vi "2_VisualizeModulePositioning2-Backup.vi"(0 "Placement Monitor":T1(plugin-control)=refnum, 1 "Calibrated positions of fiducials [mm]":dbl[][](array[numeric])=[[-658.867386146, 115.937184375, -18.342965965], [-563.38738772, 115.95451918, -18.342965965], [-563.369748267, 18.796520782, -18.342965965], [-658.849746693, 18.779185977, -18.342965965], [-560.867387761, 115.954976697, -18.342965965], [-465.387389335, 115.972311502, -18.342965965], [-465.369749882, 18.814313103, -18.342965965], [-560.849748308, 18.796978298, -18.342965965], [-462.867389377, 115.972769019, -18.342965965], [-367.38739095, 115.990103824, -18.342965965], [-367.369751497, 18.832105425, -18.342965965], [-462.849749923, 18.81477062, -18.342965965], [-364.867390992, 115.990561341, -18.342965965], [-269.387392565, 116.007896146, -18.342965965], [-269.369753112, 18.849897747, -18.342965965], [-364.849751539, 18.832562942, -18.342965965], [-266.867392607, 116.008353663, -18.342965965], [-171.38739418, 116.025688468, -18.342965965], [-171.369754727, 18.867690069, -18.342965965], [-266.849753154, 18.850355264, -18.342965965], [-168.867394222, 116.026145985, -18.342965965], [-73.387395796, 116.04348079, -18.342965965], [-73.369756342, 18.885482391, -18.342965965], [-168.849754769, 18.868147586, -18.342965965], [-70.867395837, 116.043938306, -18.342965965], [24.612602589, 116.061273111, -18.342965965], [24.630242042, 18.903274713, -18.342965965], [-70.849756384, 18.885939908, -18.342965965], [27.132602548, 116.061730628, -18.342965965], [122.612600974, 116.079065433, -18.342965965], [122.630240427, 18.921067035, -18.342965965], [27.150242001, 18.90373223, -18.342965965], [125.132600933, 116.07952295, -18.342965965], [220.612599359, 116.096857755, -18.342965965], [220.630238812, 18.938859356, -18.342965965], [125.150240386, 18.921524551, -18.342965965], [223.132599318, 116.097315272, -18.342965965], [318.612597744, 116.114650077, -18.342965965], [318.630237197, 18.956651678, -18.342965965], [223.150238771, 18.939316873, -18.342965965], [321.132597702, 116.115107594, -18.342965965], [416.612596129, 116.132442399, -18.342965965], [416.630235582, 18.974444, -18.342965965], [321.150237156, 18.957109195, -18.342965965], [419.132596087, 116.132899916, -18.342965965], [514.612594514, 116.150234721, -18.342965965], [514.630233967, 18.992236322, -18.342965965], [419.15023554, 18.974901517, -18.342965965], [517.132594472, 116.150692238, -18.342965965], [612.612592899, 116.168027043, -18.342965965], [612.630232352, 19.010028644, -18.342965965], [517.150233925, 18.992693839, -18.342965965]], 2 "XYZ .NET Refnum in":refnum<k24>, 3 "Axis Speeds":T10={"X [mm/s]"=25.0, "Y [mm/s]"=25.0, "Z [mm/s]"=25.0}, 4 "Module fiducial marker":T7=enum."Mark C", 5 "N modules":i32=13, 6 "Sensor Pattern":T8(ring)=enum."ATLAS12", 7 "error in (no error)":errorcluster, 8 "Templates path":path=path "C:/Users/Aerotech/Documents/BNL_ThermomechanicalStave", 9 "Calibration [um/pix]":dbl=1.55, 10 "Current Build Phase":refnum<vi>, 11 "Temperature":refnum<vi>, 12 "Module #":refnum<vi>, 13 "Placement tolerance [um]":dbl=25.0, 14 "Tape Type":T5=enum."Axial (Sutcliffe NP49-01-100 01-Mar-16)", 16 "Module Report":refnum<vi>, 17 "Base notes":string, 18 "Reports path":path=path "C:/Users/Aerotech/cernbox/BNL/Stave Assembly Records/2017-05-15/ModulePlacement") -> (19 "Recalibrated??":bool, 22 "XYZ .NET Refnum out":refnum<k24>, 27 "error out":errorcluster)   [LabVIEW 2016]
uses:
  Utils/Controls/All_Enums/Enum_TypeDef_FidMarkers.ctl
  C:/Users/Aerotech/Documents/BNLStaveAssembly-blueprint/Bin/Aerotech.A3200.dll
  BNLStaveAssembly-blueprint/Bin/Aerotech.A3200.dll
  Utils/Controls/All_Enums/Enum_TypeDef_CornerSelection.ctl
  Utils/Controls/All_Enums/Enum_TypeDef_TapeType.ctl
panel:
  out "Order":string[](array[string])
  out "Templates":T1[](array[plugin-control])
  out "Fiducial Template 2":T1(plugin-control)
  in  "Recalibrate!!":bool
  in  "Exit to survey or glue":bool
  out "Current task:":string="Applying glue for Module 11"
  in  "Tab Control: Positioning and Surveys":T2(tab)=enum."Apply glue"
  out "Offset interpreter":T3={"Offset Interpreter - Right"=FALSE, "Offset Interpreter - forward"=FALSE, "Offset Interpreter - backward"=TRUE, "Offset Interpreter - Left"=TRUE, "Placement Confirmation"=FALSE}
  in  "User Report: Current Module":T4={"B"=FALSE, "A"=FALSE, "D"=FALSE, "C"=FALSE, "ID"="", "Module #"=11, "x, centre"=368.8814166421462, "y, centre"=67.54477579693595, "Aligned"=FALSE, "Glue applied"=FALSE, "Placed"=FALSE}
  out "X offset [um]":sgl=497.0423
  out "Y offset [um]":sgl=417.2712
  in  "Module corner loop stop":bool
  in  "Center-only search?":bool
  in  "User notes":string="Type your note here...."
  out "Module # str":string="Module 11"
  in  "Assembly step":string(combo)
  in  "Manual Z?":bool
  in  "Manual Z [mm]":dbl
  in  "Dots (T) or Lines (F)":bool
  in  "Send XYZ Stage Away":bool
  in  "Work on Corner...":T6=enum."[Exit]"
  in  "Work on Module #...":i32=11
  in  "Tab Control":enum32{"Fiducial marker", "Error reporting"}(tab)
  out "Fiducial Template":T1(plugin-control)
  out "Mark string":string="MarkC"
  out "Current Stage Position":T9={"X [mm]"=416.6304080435383, "Y [mm]"=18.974446486493466, "Z [mm]"=-18.342965704975803}
  out "Module Progress Report":T11(array[cluster])=[{"B"=FALSE, "A"=FALSE, "D"=FALSE, "C"=FALSE, "ID"="", "Module #"=1, "x, centre"=-611.1185672065, "y, centre"=67.3668525785, "Aligned"=FALSE, "Glue applied"=FALSE, "Placed"=FALSE}, {"B"=FALSE, "A"=FALSE, "D"=FALSE, "C"=FALSE, "ID"="", "Module #"=2, "x, centre"=-513.1185688215, "y, centre"=67.3846449, "Aligned"=FALSE, "Glue applied"=FALSE, "Placed"=FALSE}, {"B"=FALSE, "A"=FALSE, "D"=FALSE, "C"=FALSE, "ID"="", "Module #"=3, "x, centre"=-415.118570437, "y, centre"=67.402437222, "Aligned"=FALSE, "Glue applied"=FALSE, "Placed"=FALSE}, {"B"=FALSE, "A"=FALSE, "D"=FALSE, "C"=FALSE, "ID"="", "Module #"=4, "x, centre"=-317.118572052, "y, centre"=67.420229544, "Aligned"=FALSE, "Glue applied"=FALSE, "Placed"=FALSE}, {"B"=FALSE, "A"=FALSE, "D"=FALSE, "C"=FALSE, "ID"="", "Module #"=5, "x, centre"=-219.118573667, "y, centre"=67.438021866, "Aligned"=FALSE, "Glue applied"=FALSE, "Placed"=FALSE}, {"B"=FALSE, "A"=FALSE, "D"=FALSE, "C"=FALSE, "ID"="", "Module #"=6, "x, centre"=-121.118575282, "y, centre"=67.455814188, "Aligned"=FALSE, "Glue applied"=FALSE, "Placed"=FALSE}, {"B"=FALSE, "A"=FALSE, "D"=FALSE, "C"=FALSE, "ID"="", "Module #"=7, "x, centre"=-23.118576897500002, "y, centre"=67.4736065095, "Aligned"=FALSE, "Glue applied"=FALSE, "Placed"=FALSE}, {"B"=FALSE, "A"=FALSE, "D"=FALSE, "C"=FALSE, "ID"="", "Module #"=8, "x, centre"=74.8814214875, "y, centre"=67.4913988315, "Aligned"=FALSE, "Glue applied"=FALSE, "Placed"=FALSE}, {"B"=FALSE, "A"=FALSE, "D"=FALSE, "C"=FALSE, "ID"="", "Module #"=9, "x, centre"=172.8814198725, "y, centre"=67.509191153, "Aligned"=FALSE, "Glue applied"=FALSE, "Placed"=FALSE}, {"B"=FALSE, "A"=FALSE, "D"=FALSE, "C"=FALSE, "ID"="", "Module #"=10, "x, centre"=270.8814182575, "y, centre"=67.52698347500001, "Aligned"=FALSE, "Glue applied"=FALSE, "Placed"=FALSE}, {"B"=FALSE, "A"=FALSE, "D"=FALSE, "C"=FALSE, "ID"="", "Module #"=11, "x, centre"=368.8814166421462, "y, centre"=67.54477579693595, "Aligned"=FALSE, "Glue applied"=FALSE, "Placed"=FALSE}, {"B"=FALSE, "A"=FALSE, "D"=FALSE, "C"=FALSE, "ID"="", "Module #"=12, "x, centre"=466.881415027, "y, centre"=67.562568119, "Aligned"=FALSE, "Glue applied"=FALSE, "Placed"=FALSE}, {"B"=FALSE, "A"=FALSE, "D"=FALSE, "C"=FALSE, "ID"="", "Module #"=13, "x, centre"=564.881413412, "y, centre"=67.580360441, "Aligned"=FALSE, "Glue applied"=FALSE, "Placed"=FALSE}]
  # "VISUALIZE MODULE PLACEMENT Brandeis University - Brookhaven National Laboratory * ATLAS Phase II Inner Tracker Upgrade * Primary Authors: Hannah Herde (hherde@brandeis.edu), Laura Bergsten (lbergsten@brandeis.edu)"
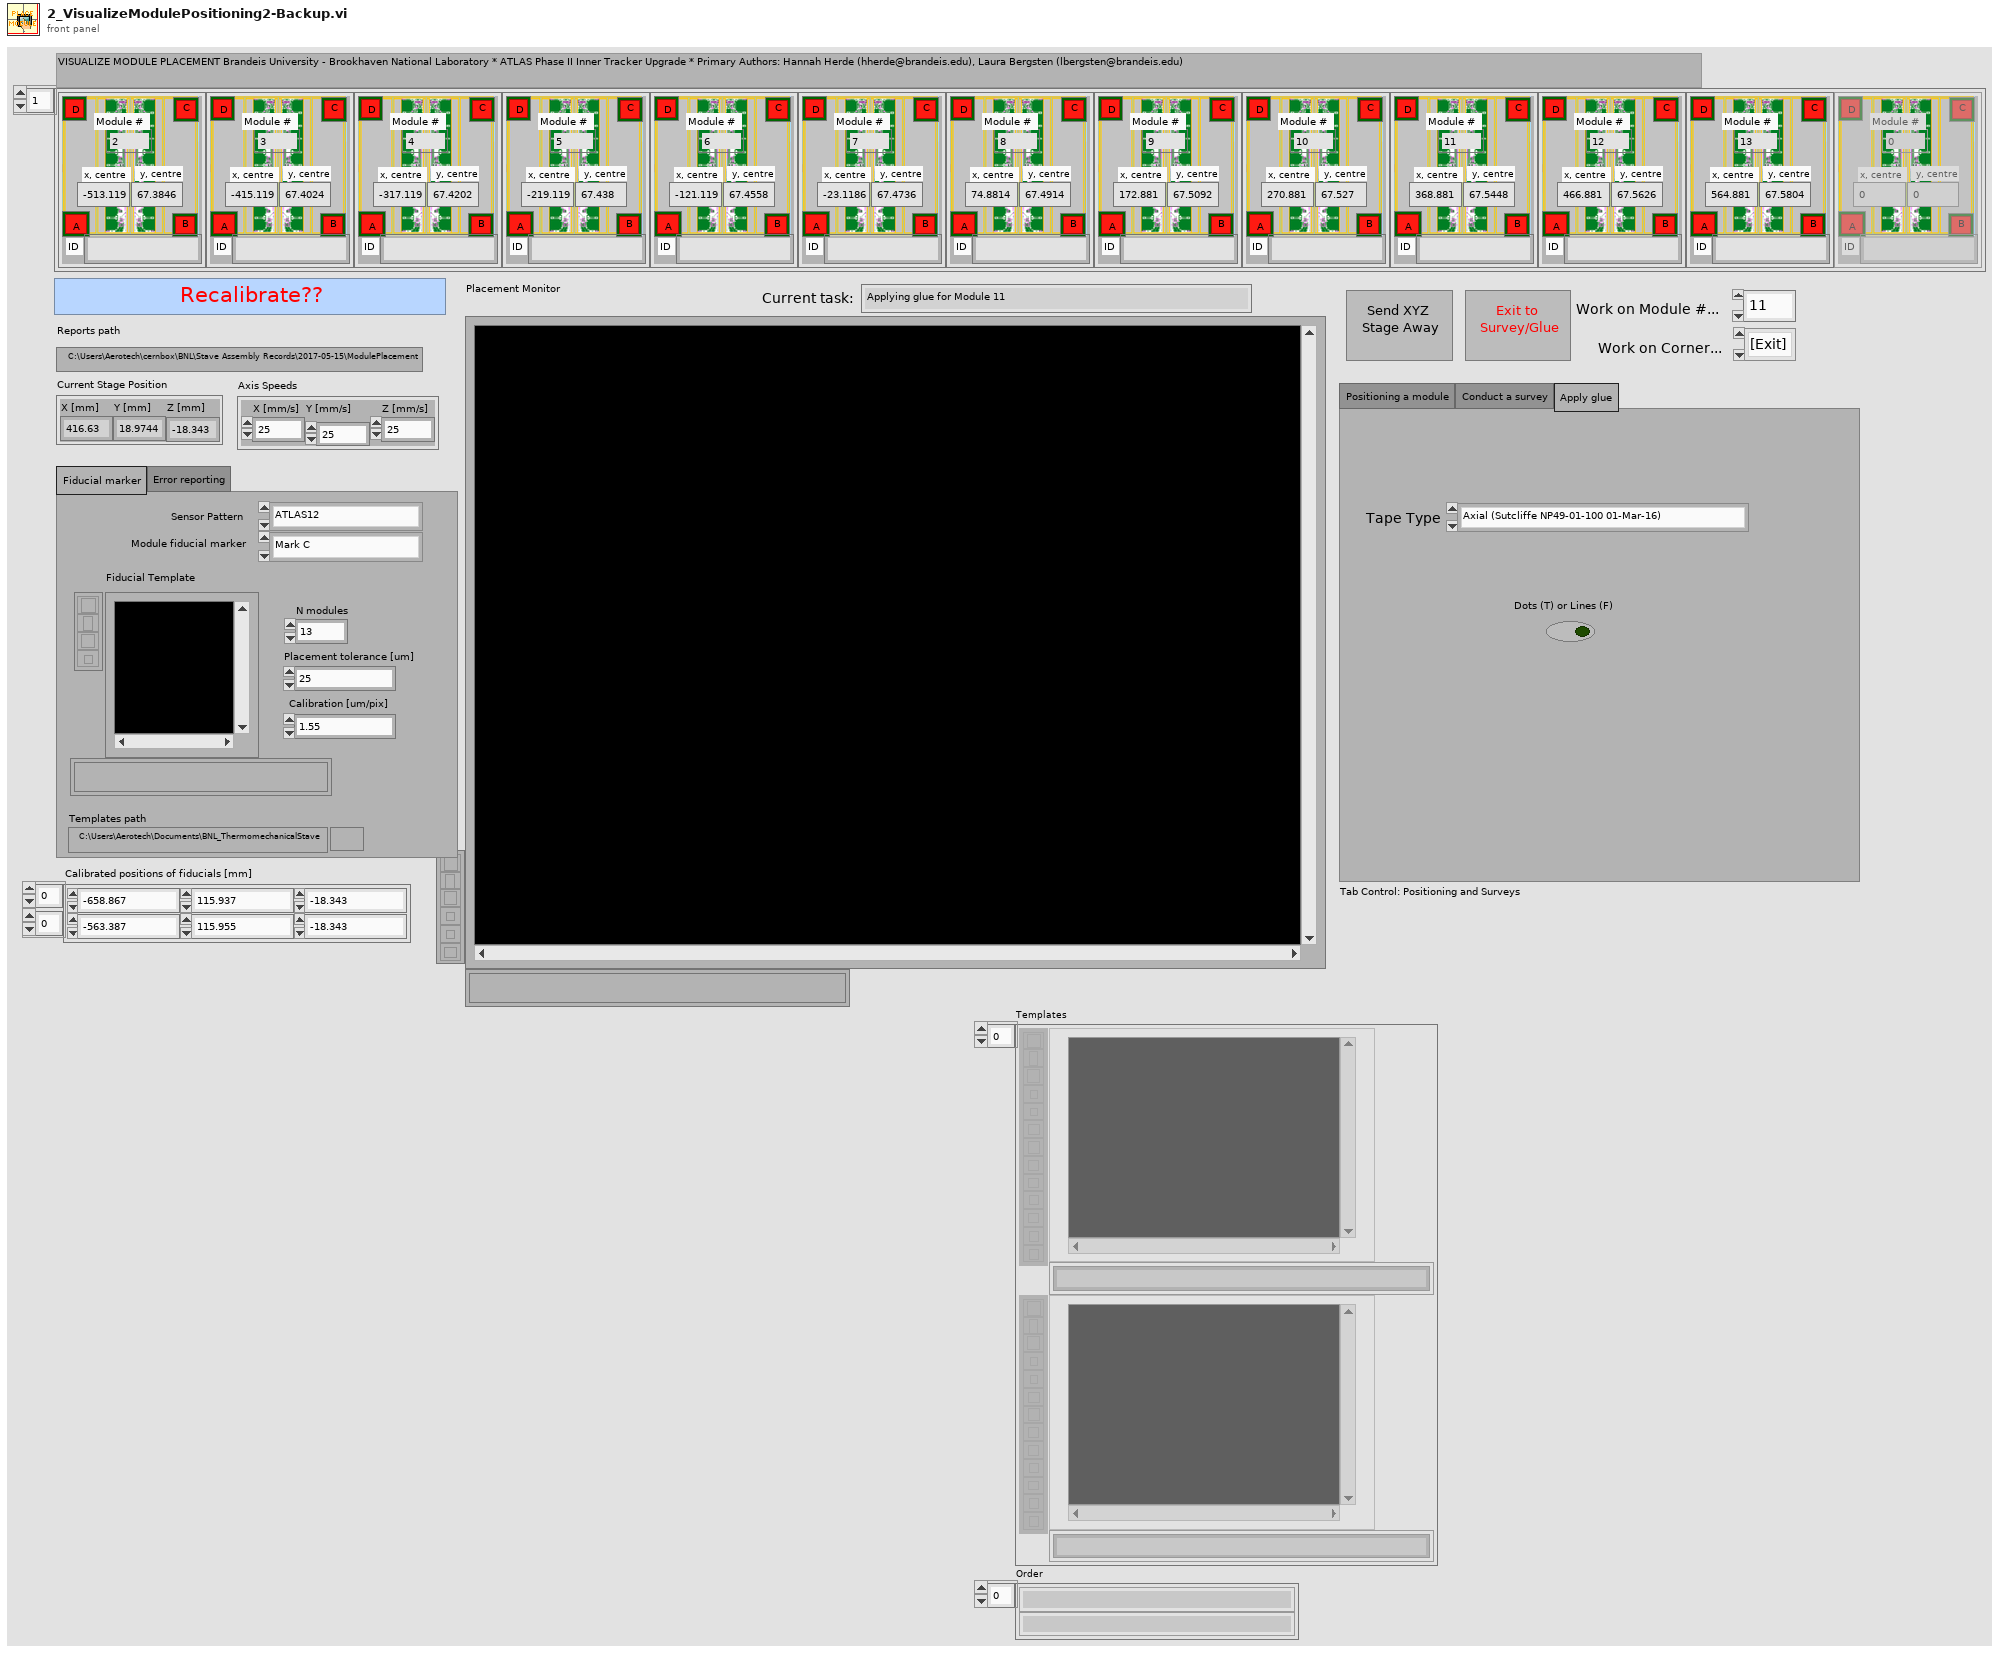
[diagram p1: front panel]
types:
  T1 = typedef "IMAQ Image.ctl" = refnum<image>
  T2 = enum32{"Positioning a module", "Conduct a survey", "Apply glue"}
  T3 = cluster{"Offset Interpreter - Right":bool, "Offset Interpreter - forward":bool, "Offset Interpreter - backward":bool, "Offset Interpreter - Left":bool, "Placement Confirmation":bool}
  T4 = cluster{"B":bool, "A":bool, "D":bool, "C":bool, "ID":string, "Module #":i32, "x, centre":dbl, "y, centre":dbl, "Aligned":bool, "Glue applied":bool, "Placed":bool}
  T5 = typedef "Enum_TypeDef_TapeType.ctl" = enum16{"Right stereo", "Left stereo", "Stereo (Sutcliffe NP49-01-100 01-Mar-16)", "Stereo (Sutcliffe 21-Jun-18- Electrical)", "Axial (Sutcliffe NP49-01-100 01-Mar-16)"}
  T6 = typedef "Enum_TypeDef_CornerSelection.ctl" = enum16{"A", "B", "C", "D", "[Exit]"}
  T7 = typedef "Enum_TypeDef_FidMarkers.ctl" = enum16{"Mark B", "Mark C", "Bias Ring Corner", "Mark I (Slim/17)", "Mark E (Slim/17)", "Mark F (Slim/17)", "Mark G (Slim/17)", "Mark A (12)", "Kapton Spacers"}
  T8 = enum16{"ATLAS07", "ATLAS12", "ATLAS12Slim", "ATLAS17LS"}
  T9 = cluster{"X [mm]":dbl, "Y [mm]":dbl, "Z [mm]":dbl}
  T10 = cluster{"X [mm/s]":dbl, "Y [mm/s]":dbl, "Z [mm/s]":dbl}
  T11 = cluster{"B":bool, "A":bool, "D":bool, "C":bool, "ID":string, "Module #":i32, "x, centre":dbl, "y, centre":dbl, "Aligned":bool, "Glue applied":bool, "Placed":bool}[]
  T12 = enum8{"Enabled", "Disabled", "Disabled and Grayed Out"}
  T13 = enum16{"Left Button", "Center Button", "Right Button", "Window Close"}
  T14 = cluster{"Final X":dbl, "Final Y":dbl, "Final Z":dbl}
  T15 = cluster{"ID":string, "Mark string":string, "Assembly step":string, "User notes":string, string, "Corner surveyed position":dbl[]}
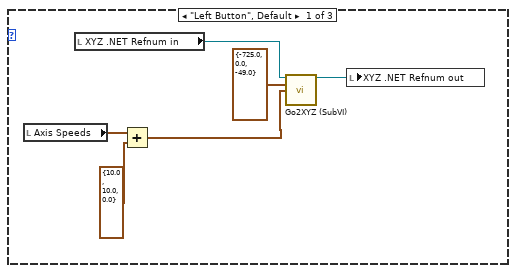
[diagram p3: hidden frame]
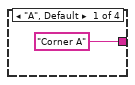
[diagram p6: hidden frame]
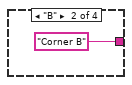
[diagram p7: hidden frame]
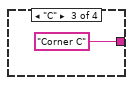
[diagram p8: hidden frame]
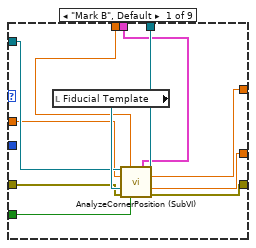
[diagram p9: hidden frame]
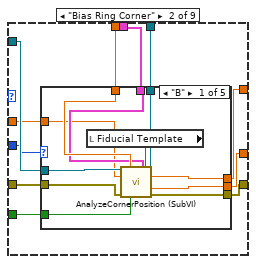
[diagram p10: hidden frame]
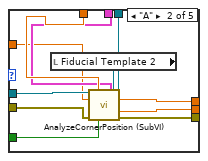
[diagram p11: hidden frame]
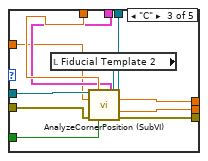
[diagram p12: hidden frame]
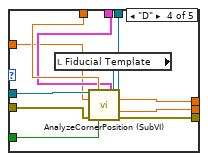
[diagram p13: hidden frame]
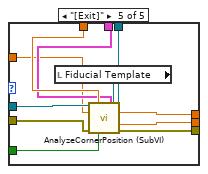
[diagram p14: hidden frame]
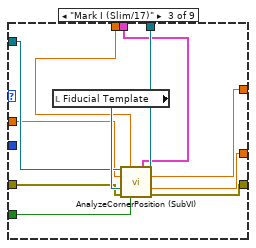
[diagram p15: hidden frame]
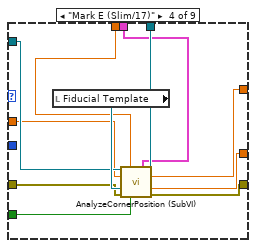
[diagram p16: hidden frame]
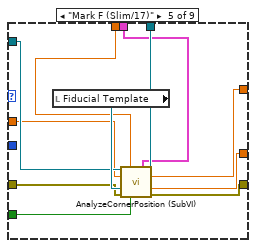
[diagram p17: hidden frame]
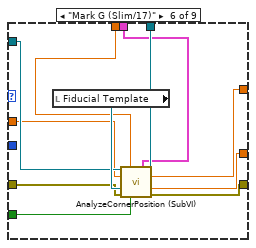
[diagram p18: hidden frame]
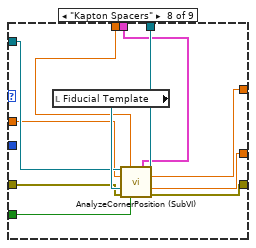
[diagram p19: hidden frame]
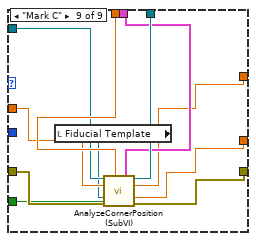
[diagram p20: hidden frame]
diagram:
  n1 = property on="Module corner loop stop" class="Bool"(error in="error in (no error)", "BoolText.Text"="Preparing..." ("Boolean Text.Text"), "DisabledEnum"=T12."Disabled and Grayed Out" ("Disabled")) -> (error out=w14:errorcluster)  [unwired: 1 in, 1 out]
  n2 = call "GetFiducialMarkTemplate (SubVI).vi"("error in (no error)"=w14, "Module fiducial marker"="Module fiducial marker", "Sensor Pattern"="Sensor Pattern", "Templates path"="Templates path") -> ("error out"=w18:errorcluster, "BiasRingCorner"=→"Fiducial Template 2":T1, "Mark string"=w3:string, "Templates"=→"Templates":T1[], "Order"=→"Order":string[])  [unwired: 3 in]
  "Mark string" <- w3
  n3 = for "Generate module placement monitor" {
    N: "N modules" -> [_]
    tunnel: "Calibrated positions of fiducials [mm]" -> [w50]
    tunnel: [w49] -> w12 mode=indexing
    tunnel: w14 -> [w30]
    tunnel: [w38] -> w5 mode=indexing
    tunnel: w3 -> [w34]
    i -> [w33]
    n4 = local read "Reports path"() -> (w32:path)
    n5 = local read "Module Progress Report"() -> (w45:T11)
    n6 = Increment(x=w33) -> (x+1=w28:i32)
    n7 = call "RecursiveDirectoryStructureGenerator (SubVI).vi"("error in (no error)"=w30, "Folder index"=w28, "Host directory"=w32) -> ("error out"=w29:errorcluster, "Nth subfolder in host directory"=w31:path)  [unwired: 7 in]
    n8 = Number To Decimal String(number=w28) -> (decimal integer string=w43:string)  [unwired: 1 in]
    n9 = Concatenate Strings("Module_" ("string"), w43, ".txt" ("string")) -> (w41:string)
    n10 = call "GetModuleReport (SubVI).vi"("error in (no error)"=w29, "Calibrated positions of fiducials [mm]"=w50, "ith Module"=w33, "Module Progress Report in"=w45) -> ("error out"=w47:errorcluster, "MyCorners"=w39:dbl[][], "Array of ith module cluster fiducial mark positions"=w49:cluster{"X":dbl, "Y":dbl, "Z":dbl}[], "Module Progress Report out"=w48:T11)  [unwired: 4 in]
    n11 = property class="Ctl"(reference="Module Report", error in=w47, "Value"=w48) -> (error out=w37:errorcluster)  [unwired: 1 out]
    n12 = Build Path(base path=w31, name or relative path=w41) -> (appended path=w35:path)
    n13 = local write "Module Progress Report"(w48) -> ()
    n14 = for {
      tunnel: string[] ["CornerA", "CornerB", "CornerC", "CornerD"] -> [w59] mode=indexing
      tunnel: w39 -> [w58] mode=indexing
      tunnel: [w57] -> w38
      tunnel: w37 -> [w56]
      tunnel: TRUE ("Write to file") -> [w55]
      tunnel: w35 -> [w54]
      tunnel: w34 -> [w53]
      n15 = call "WriteModuleToFile (SubVI).vi"("Mark used for tracking"=w53, "Assembly step"="Ideal", "User notes"="Base notes", "Current corner"=w59, "Fiducial Mark Position"=w58, "error in (no error)"=w56, "Module reports file path"=w54, "Write to file"=w55) -> ("error out"=w57:errorcluster)  [unwired: 11 in]
    }
  }
  n16 = property on="Fiducial Template" class="ImageControl"(error in=w18, "Zoom to Fit Mode"=TRUE) -> (error out=w11:errorcluster)  [unwired: 1 in, 1 out]
  n17 = property on="Module corner loop stop" class="Bool"(error in=w11, "BoolText.Text"="Preparing..." ("Boolean Text.Text"), "DisabledEnum"=T12."Disabled and Grayed Out" ("Disabled")) -> (error out=w6:errorcluster)  [unwired: 1 in, 1 out]
  n18 = Merge Errors(w6, w5) -> (w8:errorcluster)
  n19 = while {
    stop <- w60 stop-if-true
    n20 = case shown="True" "Send XYZ Stage Away" {
      frame False {
      }
      frame True {
        n21 = flat-sequence {
          frame #0 {
            n22 = call <vilib>:"Three Button Dialog.vi"("Window Title (\"\")"="Move Stage?" ("Window Title (\"\")"), "Right Button Text (\"Cancel\")"="Cancel" ("Assembly step"), "Center Button Text (\"No\")"="RIGHT" ("Assembly step"), "Left Button Text (\"Yes\")"="LEFT" ("Assembly step"), "message"="Be gone XYZ Stage" ("Assembly step")) -> ("Which Button?"=w63:T13)  [unwired: 6 in]
            n23 = case shown="\"Center Button\"" w63 {
              frame "Left Button", Default {
                n24 = local read "Axis Speeds"() -> (w70:T10)
                n25 = local read "XYZ .NET Refnum in"() -> (w73:refnum<k24>)
                n26 = Add(x=w70, y=T10 {"X [mm/s]"=10.0, "Y [mm/s]"=10.0, "Z [mm/s]"=0.0}) -> (x+y=w68:T10)
                n27 = call "Go2XYZ (SubVI).vi"(".NET Refnum in"=w73, "Go to Coordinates"=cluster{"X":dbl, "Y":dbl, "Z":dbl} {"X"=-725.0, "Y"=0.0, "Z"=-49.0}, "Axis Speeds"=w68) -> (".NET Refnum out"=w72:refnum<k24>)  [unwired: 8 in, 4 out]
                n28 = local write "XYZ .NET Refnum out"(w72) -> ()
              }
              frame "Center Button" {
                n29 = local read "Axis Speeds"() -> (w76:T10)
                n30 = local read "XYZ .NET Refnum in"() -> (w78:refnum<k24>)
                n31 = Add(x=w76, y=T10 {"X [mm/s]"=10.0, "Y [mm/s]"=10.0, "Z [mm/s]"=0.0}) -> (x+y=w74:T10)
                n32 = call "Go2XYZ (SubVI).vi"(".NET Refnum in"=w78, "Go to Coordinates"=cluster{"X":dbl, "Y":dbl, "Z":dbl} {"X"=725.0, "Y"=0.0, "Z"=-49.0}, "Axis Speeds"=w74) -> (".NET Refnum out"=w79:refnum<k24>)  [unwired: 8 in, 4 out]
                n33 = local write "XYZ .NET Refnum out"(w79) -> ()
              }
              frame "Right Button" {
              }
            }
          }
          frame #1 {
            n34 = local write "Send XYZ Stage Away"(FALSE) -> ()
          }
        }
      }
    }
    n35 = local read "Recalibrate!!"() -> (w60:bool)
  }
  n36 = while {
    tunnel: w12 -> [w93]
    shift-right: [w90] -> w7
    shift-left: w8 -> [w92]
    stop <- w87 stop-if-true
    # "Align, apply glue, and survey modules"
    n37 = local read "Recalibrate!!"() -> (w87:bool)
    "Recalibrated??" <- w87
    n38 = flat-sequence {
      tunnel: w93 -> [w99]
      tunnel: w92 -> [w97]
      tunnel: [w98] -> w91
      tunnel: [w96] -> w89
      tunnel: w87 -> [w95]
      tunnel: [w94] -> w88
      tunnel: [w393] -> w86
      tunnel: w91 -> [w393]
      tunnel: w89 -> [w392]
      tunnel: [w392] -> w84
      tunnel: w88 -> [w391]
      tunnel: [w390] -> w82
      tunnel: w86 -> [w408]
      tunnel: [w408] -> w85
      tunnel: w84 -> [w407]
      tunnel: [w407] -> w83
      tunnel: w82 -> [w406]
      tunnel: [w406] -> w81
      tunnel: w85 -> [w412]
      tunnel: [w411] -> w90
      tunnel: w83 -> [w410]
      tunnel: w81 -> [w409]
      frame #0 {
        n39 = while {
          tunnel: w99 -> [w107]
          tunnel: [w106] -> w98
          shift-right: [w104] -> w96
          shift-left: w97 -> [w103]
          tunnel: w95 -> [_]
          stop <- w102 stop-if-true
          # "Select module and corner to align"
          n40 = local read "Recalibrate!!"() -> (w101:bool)
          n41 = Equal?(x="Work on Corner...", y=enum16{"A", "B", "C", "D", "[Exit]"}."[Exit]") -> (x = y?=w110:bool)
          n42 = Or(x="Exit to survey or glue", y=w101) -> (x .or. y?=w102:bool)
          n43 = Decrement(x="Work on Module #...") -> (x-1=w108:i32)
          n44 = case shown="False" w110 {
            tunnel: "Work on Corner..." -> [w131 _]
            tunnel: w108 -> [w129 w366]
            tunnel: w107 -> [w127 w367]
            tunnel: [w121 w367] -> w106
            tunnel: "Work on Module #..." -> [w120 _]
            tunnel: w103 -> [w119 w365]
            tunnel: [w115 w363] -> w104
            frame False {
              # "Align modules"
              n45 = flat-sequence {
                tunnel: w131 -> [w132]
                tunnel: [w132] -> w130
                tunnel: w129 -> [w139]
                tunnel: [w140] -> w128
                tunnel: w127 -> [w140]
                tunnel: [w139] -> w126
                tunnel: w120 -> [w138]
                tunnel: w119 -> [w137]
                tunnel: [w136] -> w118
                tunnel: [w132] -> w113
                tunnel: w130 -> [w174]
                tunnel: w128 -> [w172]
                tunnel: w126 -> [w173]
                tunnel: [w173] -> w124
                tunnel: [w172] -> w122
                tunnel: w118 -> [w171]
                tunnel: [w170] -> w117
                tunnel: [w169] -> w114
                tunnel: w113 -> [w169]
                tunnel: [w182] -> w125
                tunnel: w124 -> [w182]
                tunnel: [w181] -> w123
                tunnel: w122 -> [w181]
                tunnel: w117 -> [w180]
                tunnel: [w179] -> w116
                tunnel: w114 -> [w178]
                tunnel: w125 -> [w357]
                tunnel: w123 -> [w356]
                tunnel: [w356] -> w121
                tunnel: w116 -> [w355]
                tunnel: [w354] -> w115
                frame #0 {
                  # "Generate labels"
                  n46 = local read "Module Progress Report"() -> (w142:T11)
                  n47 = case shown="\"D\"" w132 {
                    tunnel: ["Corner A" "Corner B" "Corner C" "Corner D"] -> w155
                    frame "A", Default {
                    }
                    frame "B" {
                    }
                    frame "C" {
                    }
                    frame "D" {
                    }
                  }
                  n48 = Empty String/Path?(string/path="Assembly step") -> (empty?=w135:bool)
                  n49 = case shown="True" w135 {
                    tunnel: [w160 "Working on" ("Assembly step")] -> w133
                    tunnel: "Assembly step" -> [w160 _]
                    frame False {
                    }
                    frame True {
                    }
                  }
                  n50 = Number To Decimal String(number=w138) -> (decimal integer string=w150:string)  [unwired: 1 in]
                  n51 = Index Array(array=w142, index=w139) -> (element=w141:T4)
                  n52 = Concatenate Strings("Module " ("string"), w150) -> (w156:string)
                  "Module # str" <- w156
                  n53 = local write "User Report: Current Module"(w141) -> ()
                  n54 = Concatenate Strings("Done with " ("string"), w156, ",  " ("string"), w155) -> (w154:string)
                  n55 = property on="Module corner loop stop" class="Bool"(error in=w137, "BoolText.Text"=w154, "DisabledEnum"=T12."Enabled" ("Disabled")) -> (error out=w159:errorcluster)  [unwired: 1 in, 1 out]
                  n56 = local read "Module Report"() -> (w143:refnum<vi>)
                  n57 = property class="Str"(reference="Module #", "Value"=w156) -> (error out=w147:errorcluster)  [unwired: 1 in, 1 out]
                  n58 = Concatenate Strings(w133, ": " ("string"), w156) -> (w148:string)
                  n59 = property class="Ctl"(reference=w143, "Value"=w142) -> (error out=w158:errorcluster)  [unwired: 1 in, 1 out]
                  n60 = property class="Str"(reference="Current Build Phase", error in=w147, "Value"=w148) -> (error out=w157:errorcluster)  [unwired: 1 out]
                  n61 = Merge Errors(w158, w157, w159) -> (w136:errorcluster)
                }
                frame #1 {
                  # "Send stage to the corner, or send it out of the way"
                  n62 = Index Array "Select a corner\non a module"(array=w172, index (row)=w173, index (col)=w174) -> (element=w167:cluster{"X":dbl, "Y":dbl, "Z":dbl})
                  n63 = call "Go2XYZ (SubVI).vi"(".NET Refnum in"="XYZ .NET Refnum in", "Go to Coordinates"=w167, "Axis Speeds"="Axis Speeds", "error in (no error)"=w171) -> (".NET Refnum out"=→"XYZ .NET Refnum out":refnum<k24>, "Final Position"=→"Current Stage Position":T14, "error out"=w170:errorcluster)  [unwired: 7 in, 2 out]
                }
                frame #2 {
                  # "Align the corner"
                  n64 = case shown="False" FALSE {
                    tunnel: w180 -> [w185 w353]
                    tunnel: [w184 w353] -> w179
                    tunnel: w178 -> [w183 _]
                    frame False {
                      n65 = while "Module Corner Placement Loop" {
                        shift-right: [w197] -> w184
                        shift-left: w185 -> [w189]
                        tunnel: w183 -> [w187]
                        stop <- "Module corner loop stop" stop-if-true
                        # "Module Corner Alignment Loop"
                        n66 = local read "Module fiducial marker"() -> (w186:T7)
                        n67 = case shown="\"Mark A (12)\"" w186 {
                          tunnel: [w207 w219 w284 w295 w306 w317 w328 w339 w352] -> w197
                          tunnel: [w203 w215 w280 w291 w302 w313 w324 w335 w351] -> w196
                          tunnel: "Placement tolerance [um]" -> [w202 w214 w279 w290 w301 w312 w323 w334 w350]
                          tunnel: "Placement Monitor" -> [w204 w216 w281 w292 w303 w314 w325 w336 w349]
                          tunnel: "Calibration [um/pix]" -> [w200 w212 w277 w288 w299 w310 w321 w332 w348]
                          tunnel: [w201 w213 w278 w289 w300 w311 w322 w333 w347] -> w192
                          tunnel: [w205 w217 w282 w293 w304 w315 w326 w337 w346] -> w191
                          tunnel: [w206 w218 w283 w294 w305 w316 w327 w338 w345] -> w190
                          tunnel: w189 -> [w208 w220 w285 w296 w307 w318 w329 w340 w344]
                          tunnel: "Center-only search?" -> [w199 w211 w276 w287 w298 w309 w320 w331 w343]
                          tunnel: w187 -> [_ w210 _ _ _ _ _ _ _]
                          frame "Mark B", Default {
                            n68 = local read "Fiducial Template"() -> (w209:T1)
                            n69 = call "AnalyzeCornerPosition (SubVI).vi"("Refnum in"=w204, "Placement tolerance [um]"=w202, "Calibration [um/pix]"=w200, "Fiducial Template"=w209, "error in (no error)"=w208, "Center-only search?"=w199) -> ("Offset interpreter"=w201:T3, "Refnum out"=w203:T1, "X offset [um]"=w205:sgl, "Y offset [um]"=w206:sgl, "error out"=w207:errorcluster)  [unwired: 3 in, 2 out]
                          }
                          frame "Bias Ring Corner" {
                            n70 = case shown="\"B\"" w210 {
                              tunnel: w220 -> [w230 w241 w252 w263 w274]
                              tunnel: [w229 w240 w251 w262 w273] -> w219
                              tunnel: [w228 w239 w250 w261 w272] -> w218
                              tunnel: [w227 w238 w249 w260 w271] -> w217
                              tunnel: w216 -> [w226 w237 w248 w259 w270]
                              tunnel: [w225 w236 w247 w258 w269] -> w215
                              tunnel: w214 -> [w224 w235 w246 w257 w268]
                              tunnel: [w223 w234 w245 w256 w267] -> w213
                              tunnel: w212 -> [w222 w233 w244 w255 w266]
                              tunnel: w211 -> [w221 w232 w243 w254 w265]
                              frame "B" {
                                n71 = local read "Fiducial Template"() -> (w231:T1)
                                n72 = call "AnalyzeCornerPosition (SubVI).vi"("Refnum in"=w226, "Placement tolerance [um]"=w224, "Calibration [um/pix]"=w222, "Fiducial Template"=w231, "error in (no error)"=w230, "Center-only search?"=w221) -> ("Offset interpreter"=w223:T3, "Refnum out"=w225:T1, "X offset [um]"=w227:sgl, "Y offset [um]"=w228:sgl, "error out"=w229:errorcluster)  [unwired: 3 in, 2 out]
                              }
                              frame "A" {
                                n73 = local read "Fiducial Template 2"() -> (w242:T1)
                                n74 = call "AnalyzeCornerPosition (SubVI).vi"("Refnum in"=w237, "Placement tolerance [um]"=w235, "Calibration [um/pix]"=w233, "Fiducial Template"=w242, "error in (no error)"=w241, "Center-only search?"=w232) -> ("Offset interpreter"=w234:T3, "Refnum out"=w236:T1, "X offset [um]"=w238:sgl, "Y offset [um]"=w239:sgl, "error out"=w240:errorcluster)  [unwired: 3 in, 2 out]
                              }
                              frame "C" {
                                n75 = local read "Fiducial Template 2"() -> (w253:T1)
                                n76 = call "AnalyzeCornerPosition (SubVI).vi"("Refnum in"=w248, "Placement tolerance [um]"=w246, "Calibration [um/pix]"=w244, "Fiducial Template"=w253, "error in (no error)"=w252, "Center-only search?"=w243) -> ("Offset interpreter"=w245:T3, "Refnum out"=w247:T1, "X offset [um]"=w249:sgl, "Y offset [um]"=w250:sgl, "error out"=w251:errorcluster)  [unwired: 3 in, 2 out]
                              }
                              frame "D" {
                                n77 = local read "Fiducial Template"() -> (w264:T1)
                                n78 = call "AnalyzeCornerPosition (SubVI).vi"("Refnum in"=w259, "Placement tolerance [um]"=w257, "Calibration [um/pix]"=w255, "Fiducial Template"=w264, "error in (no error)"=w263, "Center-only search?"=w254) -> ("Offset interpreter"=w256:T3, "Refnum out"=w258:T1, "X offset [um]"=w260:sgl, "Y offset [um]"=w261:sgl, "error out"=w262:errorcluster)  [unwired: 3 in, 2 out]
                              }
                              frame "[Exit]" {
                                n79 = local read "Fiducial Template"() -> (w275:T1)
                                n80 = call "AnalyzeCornerPosition (SubVI).vi"("Refnum in"=w270, "Placement tolerance [um]"=w268, "Calibration [um/pix]"=w266, "Fiducial Template"=w275, "error in (no error)"=w274, "Center-only search?"=w265) -> ("Offset interpreter"=w267:T3, "Refnum out"=w269:T1, "X offset [um]"=w271:sgl, "Y offset [um]"=w272:sgl, "error out"=w273:errorcluster)  [unwired: 3 in, 2 out]
                              }
                            }
                          }
                          frame "Mark I (Slim/17)" {
                            n81 = local read "Fiducial Template"() -> (w286:T1)
                            n82 = call "AnalyzeCornerPosition (SubVI).vi"("Refnum in"=w281, "Placement tolerance [um]"=w279, "Calibration [um/pix]"=w277, "Fiducial Template"=w286, "error in (no error)"=w285, "Center-only search?"=w276) -> ("Offset interpreter"=w278:T3, "Refnum out"=w280:T1, "X offset [um]"=w282:sgl, "Y offset [um]"=w283:sgl, "error out"=w284:errorcluster)  [unwired: 3 in, 2 out]
                          }
                          frame "Mark E (Slim/17)" {
                            n83 = local read "Fiducial Template"() -> (w297:T1)
                            n84 = call "AnalyzeCornerPosition (SubVI).vi"("Refnum in"=w292, "Placement tolerance [um]"=w290, "Calibration [um/pix]"=w288, "Fiducial Template"=w297, "error in (no error)"=w296, "Center-only search?"=w287) -> ("Offset interpreter"=w289:T3, "Refnum out"=w291:T1, "X offset [um]"=w293:sgl, "Y offset [um]"=w294:sgl, "error out"=w295:errorcluster)  [unwired: 3 in, 2 out]
                          }
                          frame "Mark F (Slim/17)" {
                            n85 = local read "Fiducial Template"() -> (w308:T1)
                            n86 = call "AnalyzeCornerPosition (SubVI).vi"("Refnum in"=w303, "Placement tolerance [um]"=w301, "Calibration [um/pix]"=w299, "Fiducial Template"=w308, "error in (no error)"=w307, "Center-only search?"=w298) -> ("Offset interpreter"=w300:T3, "Refnum out"=w302:T1, "X offset [um]"=w304:sgl, "Y offset [um]"=w305:sgl, "error out"=w306:errorcluster)  [unwired: 3 in, 2 out]
                          }
                          frame "Mark G (Slim/17)" {
                            n87 = local read "Fiducial Template"() -> (w319:T1)
                            n88 = call "AnalyzeCornerPosition (SubVI).vi"("Refnum in"=w314, "Placement tolerance [um]"=w312, "Calibration [um/pix]"=w310, "Fiducial Template"=w319, "error in (no error)"=w318, "Center-only search?"=w309) -> ("Offset interpreter"=w311:T3, "Refnum out"=w313:T1, "X offset [um]"=w315:sgl, "Y offset [um]"=w316:sgl, "error out"=w317:errorcluster)  [unwired: 3 in, 2 out]
                          }
                          frame "Mark A (12)" {
                            n89 = local read "Fiducial Template"() -> (w330:T1)
                            n90 = call "AnalyzeCornerPosition (SubVI).vi"("Refnum in"=w325, "Placement tolerance [um]"=w323, "Calibration [um/pix]"=w321, "Fiducial Template"=w330, "error in (no error)"=w329, "Center-only search?"=w320) -> ("Offset interpreter"=w322:T3, "Refnum out"=w324:T1, "X offset [um]"=w326:sgl, "Y offset [um]"=w327:sgl, "error out"=w328:errorcluster)  [unwired: 3 in, 2 out]
                          }
                          frame "Kapton Spacers" {
                            n91 = local read "Fiducial Template"() -> (w341:T1)
                            n92 = call "AnalyzeCornerPosition (SubVI).vi"("Refnum in"=w336, "Placement tolerance [um]"=w334, "Calibration [um/pix]"=w332, "Fiducial Template"=w341, "error in (no error)"=w340, "Center-only search?"=w331) -> ("Offset interpreter"=w333:T3, "Refnum out"=w335:T1, "X offset [um]"=w337:sgl, "Y offset [um]"=w338:sgl, "error out"=w339:errorcluster)  [unwired: 3 in, 2 out]
                          }
                          frame "Mark C" {
                            n93 = local read "Fiducial Template"() -> (w342:T1)
                            n94 = call "AnalyzeCornerPosition (SubVI).vi"("Refnum in"=w349, "Placement tolerance [um]"=w350, "Calibration [um/pix]"=w348, "Fiducial Template"=w342, "error in (no error)"=w344, "Center-only search?"=w343) -> ("Offset interpreter"=w347:T3, "Refnum out"=w351:T1, "X offset [um]"=w346:sgl, "Y offset [um]"=w345:sgl, "error out"=w352:errorcluster)  [unwired: 3 in, 2 out]
                          }
                        }
                        "X offset [um]" <- w191
                        "Y offset [um]" <- w190
                        "Offset interpreter" <- w192
                        n95 = local write "Placement Monitor"(w196) -> ()
                      }
                    }
                    frame True {
                    }
                  }
                }
                frame #3 {
                  # "Update the module progress report"
                  n96 = local read "Module Progress Report"() -> (w358:T11)
                  n97 = local read "Module Report"() -> (w361:refnum<vi>)
                  n98 = Replace Array Subset(array=w358, new element="User Report: Current Module", index=w357) -> (w359:T11)
                  n99 = property class="Ctl"(reference=w361, error in=w355, "Value"=w359) -> (error out=w354:errorcluster)  [unwired: 1 out]
                  n100 = local write "Module Progress Report"(w359) -> ()
                }
              }
            }
            frame True {
              # "Exit module alignment to do a survey or apply glue"
              n101 = disable-structure shown="Disabled" {
                disable-tunnel: w366 -> [w373 _]
                disable-tunnel: w365 -> [w369 w379]
                disable-tunnel: [w368 w378] -> w364
                frame Disabled {
                  n102 = local read "User Report: Current Module"() -> (w377:T4)
                  n103 = local read "Module Progress Report"() -> (w374:T11)
                  n104 = local read "Module Report"() -> (w376:refnum<vi>)
                  n105 = Replace Array Subset(array=w374, new element=w377, index=w373) -> (w375:T11)
                  n106 = property class="Ctl"(reference=w376, error in=w369, "Value"=w375) -> (error out=w370:errorcluster)  [unwired: 1 out]
                  n107 = local write "Module Progress Report"(w375) -> ()
                  n108 = property on="Module corner loop stop" class="Bool"(error in=w370, "BoolText.Text"="Waiting..." ("Boolean Text.Text"), "DisabledEnum"=T12."Disabled and Grayed Out" ("Disabled")) -> (error out=w368:errorcluster)  [unwired: 1 in, 1 out]
                }
                frame Enabled {
                  n109 = property on="Module corner loop stop" class="Bool"(error in=w379, "BoolText.Text"="Waiting..." ("Boolean Text.Text"), "DisabledEnum"=T12."Disabled and Grayed Out" ("Disabled")) -> (error out=w378:errorcluster)  [unwired: 1 in, 1 out]
                }
              }
              n110 = local read "Send XYZ Stage Away"() -> (w362:bool)
              n111 = case "Select destination coordinates" shown="True" w362 {
                tunnel: w364 -> [w382 w387]
                tunnel: [w382 w386] -> w363
                frame False {
                  # "Go to corner"
                }
                frame True {
                  # "Send stage away"
                  n112 = local read "XYZ .NET Refnum in"() -> (w384:refnum<k24>)
                  n113 = local read "Axis Speeds"() -> (w388:T10)
                  n114 = call "Go2XYZ (SubVI).vi"(".NET Refnum in"=w384, "Go to Coordinates"=cluster{"X":dbl, "Y":dbl, "Z":dbl} {"X"=-725.0, "Y"=0.0, "Z"=-49.0}, "Axis Speeds"=w388, "error in (no error)"=w387) -> (".NET Refnum out"=w385:refnum<k24>, "Final Position"=w383:T14, "error out"=w386:errorcluster)  [unwired: 7 in, 2 out]
                  n115 = local write "XYZ .NET Refnum out"(w385) -> ()
                  n116 = local write "Current Stage Position"(w383) -> ()
                }
              }
            }
          }
          "Current task:" <- "Aligning modules..." ("Prgm dialogue")
        }
        n117 = local read "Exit to survey or glue"() -> (w94:bool)
      }
      frame #1 {
        n118 = case shown="True" w391 {
          tunnel: [T13."Right Button" ("Which Button?") w402] -> w390
          frame False {
          }
          frame True {
            n119 = local read "Assembly step"() -> (w398:string)
            n120 = local read "Module # str"() -> (w401:string)
            n121 = local write "Exit to survey or glue"(FALSE ("Exit to survey or glue")) -> ()
            n122 = Concatenate Strings("Would you like to survey or glue " ("message"), w401, "? Survey results will be labeled \"" ("string"), w398, ".\"" ("string")) -> (w396:string)
            n123 = call <vilib>:"Three Button Dialog.vi"("Right Button Text (\"Cancel\")"="Cancel" ("Right Button Text (\"Cancel\")"), "Center Button Text (\"No\")"="Apply glue" ("Center Button Text (\"No\")"), "Left Button Text (\"Yes\")"="Survey" ("Left Button Text (\"Yes\")"), "message"=w396) -> ("Which Button?"=w402:T13)  [unwired: 7 in]
          }
        }
      }
      frame #2 {
      }
      frame #3 {
        n124 = case shown="\"Left Button\"" w409 {
          tunnel: w412 -> [w434 w631 _]
          tunnel: [w422 w632 w685] -> w411
          tunnel: w410 -> [w418 w630 w685]
          frame "Left Button" {
            # "Do a survey"
            n125 = local read "Module # str"() -> (w414:string)
            n126 = local read "Work on Module #..."() -> (w416:i32)
            n127 = local read "Module Progress Report"() -> (w427:T11)
            n128 = Concatenate Strings("Surveying " ("Prgm dialogue"), w414) -> (w413:string)
            n129 = Number To Decimal String(number=w416) -> (decimal integer string=w435:string)  [unwired: 1 in]
            n130 = Decrement(x=w416) -> (x-1=w419:i32)
            n131 = local write "Current task:"(w413) -> ()
            n132 = call "RecursiveDirectoryStructureGenerator (SubVI).vi"("error in (no error)"=w418, "Folder index"=w416, "Host directory"="Reports path") -> ("error out"=w417:errorcluster, "Nth subfolder in host directory"=w421:path)  [unwired: 7 in]
            n133 = Index Array(array=w427, index=w419) -> (element=w425:T4)
            n134 = Concatenate Strings("Module_" ("string"), w435) -> (w423:string)
            n135 = Index Array(array=w434, index (row)=w419) -> (element=w436:cluster{"X":dbl, "Y":dbl, "Z":dbl}[])  [unwired: 1 in]
            n136 = for "Survey and save a corner of the module" {
              tunnel: w421 -> [w462]
              tunnel: [w475] -> w433 mode=indexing
              tunnel: w436 -> [w447] mode=indexing
              tunnel: string[] ["A", "B", "C", "D"] -> [w443] mode=indexing
              tunnel: w425 -> [w469]
              tunnel: w423 -> [w450]
              tunnel: w417 -> [w449]
              w452 = "_" ("string")
              n137 = local read "Placement tolerance [um]"() -> (w473:dbl)
              n138 = local read "Module fiducial marker"() -> (w445:T7)
              n139 = local read "Manual Z?"() -> (w446:bool)
              n140 = local read "Calibration [um/pix]"() -> (w472:dbl)
              n141 = local read "XYZ .NET Refnum in"() -> (w478:refnum<k24>)
              n142 = local read "Axis Speeds"() -> (w471:T10)
              n143 = local read "Placement Monitor"() -> (w474:T1)
              n144 = Unbundle By Name(w469) -> ("ID"=w468:string)
              n145 = Concatenate Strings(w450, ".txt" ("string")) -> (w464:string)
              n146 = local read "Assembly step"() -> (w451:string)
              n147 = case shown="True" w446 {
                tunnel: w447 -> [w622 w627]
                tunnel: [w622 w623] -> w448
                frame False {
                }
                frame True {
                  n148 = local read "Manual Z [mm]"() -> (w624:dbl)
                  n149 = Unbundle By Name(w627) -> ("X"=w626:dbl, "Y"=w625:dbl)
                  n150 = Bundle("X"=w626, "Y"=w625, "Manual Z [mm]"=w624) -> (w623:cluster{"X":dbl, "Y":dbl, "Manual Z [mm]":dbl})  [unwired: 1 in]
                }
              }
              n151 = Equal?(x=w443, y="A") -> (x = y?=w440:bool)
              n152 = Equal?(x=w443, y="C") -> (x = y?=w441:bool)
              n153 = Build Path(base path=w462, name or relative path=w464) -> (appended path=w463:path)
              n154 = Concatenate Strings("Corner" ("string"), w443) -> (w460:string)
              n155 = Or(x=w440, y=w441) -> (x .or. y?=w439:bool)
              n156 = case shown="\"Mark I (Slim/17)\"" w445 {
                tunnel: w478 -> [w491 w504 w517 w556 w569 w582 w595 w608 w621]
                tunnel: [w489 w502 w516 w554 w567 w580 w593 w606 w619] -> w476
                tunnel: w474 -> [w488 w501 w515 w553 w566 w579 w592 w605 w618]
                tunnel: w473 -> [w487 w500 w514 w552 w565 w578 w591 w604 w617]
                tunnel: w472 -> [w486 w499 w513 w551 w564 w577 w590 w603 w616]
                tunnel: w471 -> [w485 w498 w512 w550 w563 w576 w589 w602 w615]
                tunnel: [w484 w497 w511 w549 w562 w575 w588 w601 w614] -> w457
                tunnel: [w483 w496 w510 w548 w561 w574 w587 w600 w613] -> w455
                tunnel: [w482 w495 w509 w547 w560 w573 w586 w599 w612] -> w454
                tunnel: [w481 w494 w508 w546 w559 w572 w585 w598 w611] -> w453
                tunnel: w449 -> [w480 w493 w507 w545 w558 w571 w584 w597 w610]
                tunnel: w448 -> [w479 w492 w506 w544 w557 w570 w583 w596 w609]
                tunnel: w439 -> [_ _ w505 _ _ _ _ _ _]
                frame "Mark C", Default {
                  n157 = local read "Fiducial Template"() -> (w490:T1)
                  n158 = call "CollectCorner (SubVI).vi"("XYZ .NET Refnum in"=w491, "Calibration [um/pix]"=w486, "Placement tolerance [um]"=w487, "Placement Monitor"=w488, "Fiducial Template"=w490, "error in (no error)"=w480, "Axis Speeds"=w485, "Corner Coordinates"=w479) -> ("XYZ .NET Refnum out"=w481:refnum<k24>, "Placement Monitor out"=w482:T1, "Corner surveyed position"=w484:dbl[], "XYZ Stage Final Position"=w483:T14, "error out"=w489:errorcluster)  [unwired: 3 in]
                }
                frame "Mark B" {
                  n159 = local read "Fiducial Template"() -> (w503:T1)
                  n160 = call "CollectCorner (SubVI).vi"("XYZ .NET Refnum in"=w504, "Calibration [um/pix]"=w499, "Placement tolerance [um]"=w500, "Placement Monitor"=w501, "Fiducial Template"=w503, "error in (no error)"=w493, "Axis Speeds"=w498, "Corner Coordinates"=w492) -> ("XYZ .NET Refnum out"=w494:refnum<k24>, "Placement Monitor out"=w495:T1, "Corner surveyed position"=w497:dbl[], "XYZ Stage Final Position"=w496:T14, "error out"=w502:errorcluster)  [unwired: 3 in]
                }
                frame "Bias Ring Corner" {
                  n161 = case shown="True" w505 {
                    tunnel: w517 -> [w530 w543]
                    tunnel: [w528 w541] -> w516
                    tunnel: w515 -> [w527 w540]
                    tunnel: w514 -> [w526 w539]
                    tunnel: w513 -> [w525 w538]
                    tunnel: w512 -> [w524 w537]
                    tunnel: [w523 w536] -> w511
                    tunnel: [w522 w535] -> w510
                    tunnel: [w521 w534] -> w509
                    tunnel: [w520 w533] -> w508
                    tunnel: w507 -> [w519 w532]
                    tunnel: w506 -> [w518 w531]
                    frame True {
                      n162 = local read "Fiducial Template 2"() -> (w529:T1)
                      n163 = call "CollectCorner (SubVI).vi"("XYZ .NET Refnum in"=w530, "Calibration [um/pix]"=w525, "Placement tolerance [um]"=w526, "Placement Monitor"=w527, "Fiducial Template"=w529, "error in (no error)"=w519, "Axis Speeds"=w524, "Corner Coordinates"=w518) -> ("XYZ .NET Refnum out"=w520:refnum<k24>, "Placement Monitor out"=w521:T1, "Corner surveyed position"=w523:dbl[], "XYZ Stage Final Position"=w522:T14, "error out"=w528:errorcluster)  [unwired: 3 in]
                    }
                    frame False {
                      n164 = local read "Fiducial Template"() -> (w542:T1)
                      n165 = call "CollectCorner (SubVI).vi"("XYZ .NET Refnum in"=w543, "Calibration [um/pix]"=w538, "Placement tolerance [um]"=w539, "Placement Monitor"=w540, "Fiducial Template"=w542, "error in (no error)"=w532, "Axis Speeds"=w537, "Corner Coordinates"=w531) -> ("XYZ .NET Refnum out"=w533:refnum<k24>, "Placement Monitor out"=w534:T1, "Corner surveyed position"=w536:dbl[], "XYZ Stage Final Position"=w535:T14, "error out"=w541:errorcluster)  [unwired: 3 in]
                    }
                  }
                }
                frame "Mark I (Slim/17)" {
                  n166 = local read "Fiducial Template"() -> (w555:T1)
                  n167 = call "CollectCorner (SubVI).vi"("XYZ .NET Refnum in"=w556, "Calibration [um/pix]"=w551, "Placement tolerance [um]"=w552, "Placement Monitor"=w553, "Fiducial Template"=w555, "error in (no error)"=w545, "Axis Speeds"=w550, "Corner Coordinates"=w544) -> ("XYZ .NET Refnum out"=w546:refnum<k24>, "Placement Monitor out"=w547:T1, "Corner surveyed position"=w549:dbl[], "XYZ Stage Final Position"=w548:T14, "error out"=w554:errorcluster)  [unwired: 3 in]
                }
                frame "Mark E (Slim/17)" {
                  n168 = local read "Fiducial Template"() -> (w568:T1)
                  n169 = call "CollectCorner (SubVI).vi"("XYZ .NET Refnum in"=w569, "Calibration [um/pix]"=w564, "Placement tolerance [um]"=w565, "Placement Monitor"=w566, "Fiducial Template"=w568, "error in (no error)"=w558, "Axis Speeds"=w563, "Corner Coordinates"=w557) -> ("XYZ .NET Refnum out"=w559:refnum<k24>, "Placement Monitor out"=w560:T1, "Corner surveyed position"=w562:dbl[], "XYZ Stage Final Position"=w561:T14, "error out"=w567:errorcluster)  [unwired: 3 in]
                }
                frame "Mark F (Slim/17)" {
                  n170 = local read "Fiducial Template"() -> (w581:T1)
                  n171 = call "CollectCorner (SubVI).vi"("XYZ .NET Refnum in"=w582, "Calibration [um/pix]"=w577, "Placement tolerance [um]"=w578, "Placement Monitor"=w579, "Fiducial Template"=w581, "error in (no error)"=w571, "Axis Speeds"=w576, "Corner Coordinates"=w570) -> ("XYZ .NET Refnum out"=w572:refnum<k24>, "Placement Monitor out"=w573:T1, "Corner surveyed position"=w575:dbl[], "XYZ Stage Final Position"=w574:T14, "error out"=w580:errorcluster)  [unwired: 3 in]
                }
                frame "Mark G (Slim/17)" {
                  n172 = local read "Fiducial Template"() -> (w594:T1)
                  n173 = call "CollectCorner (SubVI).vi"("XYZ .NET Refnum in"=w595, "Calibration [um/pix]"=w590, "Placement tolerance [um]"=w591, "Placement Monitor"=w592, "Fiducial Template"=w594, "error in (no error)"=w584, "Axis Speeds"=w589, "Corner Coordinates"=w583) -> ("XYZ .NET Refnum out"=w585:refnum<k24>, "Placement Monitor out"=w586:T1, "Corner surveyed position"=w588:dbl[], "XYZ Stage Final Position"=w587:T14, "error out"=w593:errorcluster)  [unwired: 3 in]
                }
                frame "Mark A (12)" {
                  n174 = local read "Fiducial Template"() -> (w607:T1)
                  n175 = call "CollectCorner (SubVI).vi"("XYZ .NET Refnum in"=w608, "Calibration [um/pix]"=w603, "Placement tolerance [um]"=w604, "Placement Monitor"=w605, "Fiducial Template"=w607, "error in (no error)"=w597, "Axis Speeds"=w602, "Corner Coordinates"=w596) -> ("XYZ .NET Refnum out"=w598:refnum<k24>, "Placement Monitor out"=w599:T1, "Corner surveyed position"=w601:dbl[], "XYZ Stage Final Position"=w600:T14, "error out"=w606:errorcluster)  [unwired: 3 in]
                }
                frame "Kapton Spacers" {
                  n176 = local read "Fiducial Template"() -> (w620:T1)
                  n177 = call "CollectCorner (SubVI).vi"("XYZ .NET Refnum in"=w621, "Calibration [um/pix]"=w616, "Placement tolerance [um]"=w617, "Placement Monitor"=w618, "Fiducial Template"=w620, "error in (no error)"=w610, "Axis Speeds"=w615, "Corner Coordinates"=w609) -> ("XYZ .NET Refnum out"=w611:refnum<k24>, "Placement Monitor out"=w612:T1, "Corner surveyed position"=w614:dbl[], "XYZ Stage Final Position"=w613:T14, "error out"=w619:errorcluster)  [unwired: 3 in]
                }
              }
              n178 = local read "Mark string"() -> (w467:string)
              n179 = Concatenate Strings(w450, w452, w451, w452, w460, ".png" ("string")) -> (w459:string)
              n180 = Bundle("ID"=w468, "Mark string"=w467, "Assembly step"=w451, "User notes"="User notes", w460, "Corner surveyed position"=w457) -> (w456:T15)  [unwired: 1 in]
              n181 = Build Path(base path=w462, name or relative path=w459) -> (appended path=w458:path)
              n182 = local write "Placement Monitor"(w454) -> ()
              n183 = local write "XYZ .NET Refnum out"(w453) -> ()
              n184 = local write "Current Stage Position"(w455) -> ()
              n185 = property class="Slide (strict)"(reference="Temperature") -> ("Value"=w437:dbl)  [unwired: 1 in, 2 out]
              n186 = call "SaveCorner (SubVI).vi"("Module record filename"=w463, "Temperature"=w437, "Write to file"=TRUE, "Data strings"=w456, "Module corner image filename"=w458, "Image of corner"=w454, "error in (no error)"=w476) -> ("error out"=w475:errorcluster)  [unwired: 8 in]
            }
            n187 = local read "User Report: Current Module"() -> (w432:T4)
            n188 = local read "Module Progress Report"() -> (w429:T11)
            n189 = Replace Array Subset(array=w429, new element=w432, index=w419) -> (w430:T11)
            n190 = local write "Module Progress Report"(w430) -> ()
            n191 = local read "Module Report"() -> (w431:refnum<vi>)
            n192 = Merge Errors(w433) -> (w428:errorcluster)
            n193 = property class="Ctl"(reference=w431, error in=w428, "Value"=w430) -> (error out=w422:errorcluster)  [unwired: 1 out]
          }
          frame "Center Button" {
            # "Apply Glue"
            n194 = Two Button Dialog(message="Are you sure?" ("Center Button Text (\"No\")")) -> (T button?=w628:bool)  [unwired: 2 in]
            n195 = case shown="True" w628 {
              tunnel: [w633 w664] -> w632
              tunnel: w631 -> [_ w662]
              tunnel: w630 -> [w633 w659]
              frame False {
              }
              frame True {
                # "Apply glue lives here"
                n196 = local read "Work on Module #..."() -> (w645:i32)
                n197 = local read "Module # str"() -> (w639:string)
                n198 = Decrement(x=w645) -> (x-1=w663:i32)
                n199 = Concatenate Strings("Applying glue for " ("Prgm dialogue"), w639) -> (w638:string)
                n200 = Index Array(array=w662, index (row)=w663) -> (element=w661:cluster{"X":dbl, "Y":dbl, "Z":dbl}[])  [unwired: 1 in]
                n201 = local write "Current task:"(w638) -> ()
                n202 = for {
                  tunnel: w661 -> [w684] mode=indexing
                  tunnel: [w683] -> w660 mode=indexing
                  n203 = Cluster To Array(cluster=w684) -> (array=w683:dbl[])
                }
                n204 = local read "Reports path"() -> (w646:path)
                n205 = call "GetModuleCentre (SubVI).vi"("error in (no error)"=w659, "4x3 Array of Fiducial Coordinates"=w660) -> ("error out"=w644:errorcluster, "y, centre"=w655:dbl, "x, centre"=w658:dbl)  [unwired: 1 in]
                n206 = call "RecursiveDirectoryStructureGenerator (SubVI).vi"("error in (no error)"=w644, "Folder index"=w645, "Host directory"=w646) -> ("error out"=w643:errorcluster, "Nth subfolder in host directory"=w635:path)  [unwired: 7 in]
                n207 = Add(x=w655, y=42.5) -> (x+y=w652:dbl)
                n208 = Add(x=w658, y=-42.5) -> (x+y=w653:dbl)
                n209 = local read "Templates path"() -> (w641:path)
                n210 = local read "XYZ .NET Refnum in"() -> (w649:refnum<k24>)
                n211 = local read "Calibration [um/pix]"() -> (w654:dbl)
                n212 = local read "Placement Monitor"() -> (w647:T1)
                n213 = Bundle(w653, w652, "y"=-49.0) -> (w650:cluster{dbl, dbl, "y":dbl})  [unwired: 1 in]
                n214 = Build Path(base path=w641, name or relative path="Utils\\ConfigurationFiles_and_Templates\\1_ModulePlacement") -> (appended path=w640:path)
                n215 = case shown="False" "Dots (T) or Lines (F)" {
                  tunnel: [w666 w682] -> w664
                  tunnel: w654 -> [w672 w681]
                  tunnel: w650 -> [w670 w680]
                  tunnel: w649 -> [w669 w679]
                  tunnel: [w668 w678] -> w648
                  tunnel: w647 -> [w667 w677]
                  tunnel: w643 -> [w671 w676]
                  tunnel: w640 -> [w665 w675]
                  tunnel: "Tape Type" -> [_ w674]
                  tunnel: w635 -> [_ w673]
                  frame False {
                    n216 = call "LauraMod_GlueFatLines.vi"("Image Feed"=w667, "Template Path"=w665, "error in"=w671, "um/pix resolution"=w672, "Module corner coordinates"=w670, "XYZ Stage Control"=w669) -> ("error out"=w666:errorcluster, "XYZ .NET Refnum out"=w668:refnum<k24>)  [unwired: 4 in]
                  }
                  frame True {
                    n217 = call "GlueSingleModule(SubVI).vi"("XYZ Stage Control"=w679, "Template Path"=w675, "Image Feed"=w677, "Module corner coordinates"=w680, "Path to save collected images"=w673, "um/pix resolution"=w681, "error in"=w676, "Tape Type"=w674) -> ("XYZ .NET Refnum out"=w678:refnum<k24>, "error out"=w682:errorcluster)  [unwired: 6 in]
                  }
                }
                n218 = local write "XYZ .NET Refnum out"(w648) -> ()
              }
            }
          }
          frame "Right Button", Default {
            # "Do nothing -- go back to positioning modules"
            # "Do nothing (exit or return to module alignment)"
          }
        }
      }
    }
  }
  n219 = local read "Fiducial Template"() -> (w27:T1)
  n220 = call "IMAQ Dispose"("Image"=w27, "error in (no error)"=w7) -> ("error out"=w26:errorcluster)  [unwired: 4 in]
  n221 = call <vilib>:"General Error Handler.vi"("error in (no error)"=w26) -> ("error out"=→"error out":errorcluster)  [unwired: 10 in, 4 out]
  "Module Progress Report" <- T11 [] ("Module Progress Report")
